vi "Dresden R2R Sputter 03.02.2018 IY24.vi"() -> ()   [LabVIEW 2009] (continued)
                                frame #0 {
                                n30316 = local write "SDC1 9"(TRUE ("SDC1 9")) -> ()
                                n30317 = Wait (ms)(milliseconds to wait=u32 1000) -> ()  [unwired: 1 out]
                                }
                                frame #1 {
                                }
                                }
                                }
                                }
                                }
                                }
                                }
                                frame #1 {
                                }
                                }
                                }
                                frame #11 {
                                n30318 = local read "Semi"() -> (w35192:bool)
                                n30319 = case shown="False" w35192 {
                                frame #0 {
                                n30320 = local write "Start_roll"(TRUE ("Start_roll")) -> ()
                                n30321 = Wait (ms)(milliseconds to wait=u32 300) -> ()  [unwired: 1 out]
                                }
                                frame #1 {
                                }
                                }
                                }
                                frame #12 {
                                n30322 = local read "Semi"() -> (w35195:bool)
                                n30323 = case shown="False" w35195 {
                                frame #0 {
                                n30324 = stacked-sequence {
                                frame #0 {
                                n30325 = local read "R Cmb Ch2 Step1 Coating Power Active"() -> (w35196:bool)
                                n30326 = case shown="True" w35196 {
                                frame #0 {
                                }
                                frame #1 {
                                n30327 = while {
                                stop <- w35198 stop-if-true
                                n30328 = local read "R Cmb Interval length"() -> (w35202:dbl)
                                n30329 = local read "Actual Length"() -> (w35201:dbl)
                                n30330 = Greater Or Equal?(x=w35201, y=w35202) -> (x >= y?=w35200:bool)
                                n30331 = local read "Semi"() -> (w35199:bool)
                                n30332 = Or(x=w35200, y=w35199) -> (x .or. y?=w35198:bool)
                                n30333 = Wait Until Next ms Multiple(millisecond multiple=u32 300) -> ()  [unwired: 1 out]
                                }
                                }
                                }
                                }
                                frame #1 {
                                n30334 = local read "R Cmb Ch2 Step2 Coating Power Active"() -> (w35203:bool)
                                n30335 = case shown="True" w35203 {
                                frame #0 {
                                }
                                frame #1 {
                                n30336 = stacked-sequence {
                                frame #0 {
                                n30337 = local read "Semi"() -> (w35204:bool)
                                n30338 = case shown="False" w35204 {
                                frame #0 {
                                n30339 = local read "R Cmb Ch3 Step2 Coating Power"() -> (w35206:dbl)
                                n30340 = Wait (ms)(milliseconds to wait=u32 200) -> ()  [unwired: 1 out]
                                n30341 = local write "Set DC Power       : 2"(w35206) -> ()
                                }
                                frame #1 {
                                }
                                }
                                }
                                frame #1 {
                                n30342 = local read "Semi"() -> (w35207:bool)
                                n30343 = case shown="False" w35207 {
                                frame #0 {
                                n30344 = local write "Dc_auto_set"(TRUE ("Dc_auto_set")) -> ()
                                }
                                frame #1 {
                                }
                                }
                                }
                                frame #2 {
                                n30345 = while {
                                stop <- w35213 stop-if-true
                                n30346 = local read "R Cmb Interval length"() -> (w35212:dbl)
                                n30347 = local read "Actual Length"() -> (w35216:dbl)
                                n30348 = Multiply(x=w35212, y=2.0) -> (x*y=w35210:dbl)
                                n30349 = Greater Or Equal?(x=w35216, y=w35210) -> (x >= y?=w35215:bool)
                                n30350 = local read "Semi"() -> (w35214:bool)
                                n30351 = Or(x=w35215, y=w35214) -> (x .or. y?=w35213:bool)
                                n30352 = Wait Until Next ms Multiple(millisecond multiple=u32 300) -> ()  [unwired: 1 out]
                                }
                                }
                                }
                                }
                                }
                                }
                                frame #2 {
                                n30353 = local read "R Cmb Ch2 Step3 Coating Power Active"() -> (w35217:bool)
                                n30354 = case shown="True" w35217 {
                                frame #0 {
                                }
                                frame #1 {
                                n30355 = stacked-sequence {
                                frame #0 {
                                n30356 = local read "Semi"() -> (w35218:bool)
                                n30357 = case shown="False" w35218 {
                                frame #0 {
                                n30358 = local read "R Cmb Ch3 Step3 Coating Power"() -> (w35220:dbl)
                                n30359 = Wait (ms)(milliseconds to wait=u32 200) -> ()  [unwired: 1 out]
                                n30360 = local write "Set DC Power       : 2"(w35220) -> ()
                                }
                                frame #1 {
                                }
                                }
                                }
                                frame #1 {
                                n30361 = local read "Semi"() -> (w35221:bool)
                                n30362 = case shown="False" w35221 {
                                frame #0 {
                                n30363 = local write "Dc_auto_set"(TRUE ("Dc_auto_set")) -> ()
                                }
                                frame #1 {
                                }
                                }
                                }
                                frame #2 {
                                n30364 = while {
                                stop <- w35227 stop-if-true
                                n30365 = local read "R Cmb Interval length"() -> (w35226:dbl)
                                n30366 = local read "Actual Length"() -> (w35230:dbl)
                                n30367 = Multiply(x=w35226, y=3.0) -> (x*y=w35224:dbl)
                                n30368 = Greater Or Equal?(x=w35230, y=w35224) -> (x >= y?=w35229:bool)
                                n30369 = local read "Semi"() -> (w35228:bool)
                                n30370 = Or(x=w35229, y=w35228) -> (x .or. y?=w35227:bool)
                                n30371 = Wait Until Next ms Multiple(millisecond multiple=u32 300) -> ()  [unwired: 1 out]
                                }
                                }
                                }
                                }
                                }
                                }
                                frame #3 {
                                n30372 = local read "R Cmb Ch2 Step4 Coating Power Active"() -> (w35231:bool)
                                n30373 = case shown="True" w35231 {
                                frame #0 {
                                }
                                frame #1 {
                                n30374 = stacked-sequence {
                                frame #0 {
                                n30375 = local read "Semi"() -> (w35232:bool)
                                n30376 = case shown="False" w35232 {
                                frame #0 {
                                n30377 = local read "R Cmb Ch3 Step4 Coating Power"() -> (w35234:dbl)
                                n30378 = Wait (ms)(milliseconds to wait=u32 200) -> ()  [unwired: 1 out]
                                n30379 = local write "Set DC Power       : 2"(w35234) -> ()
                                }
                                frame #1 {
                                }
                                }
                                }
                                frame #1 {
                                n30380 = local read "Semi"() -> (w35235:bool)
                                n30381 = case shown="False" w35235 {
                                frame #0 {
                                n30382 = local write "Dc_auto_set"(TRUE ("Dc_auto_set")) -> ()
                                }
                                frame #1 {
                                }
                                }
                                }
                                frame #2 {
                                n30383 = while {
                                stop <- w35241 stop-if-true
                                n30384 = local read "R Cmb Interval length"() -> (w35240:dbl)
                                n30385 = local read "Actual Length"() -> (w35244:dbl)
                                n30386 = Multiply(x=w35240, y=4.0) -> (x*y=w35238:dbl)
                                n30387 = Greater Or Equal?(x=w35244, y=w35238) -> (x >= y?=w35243:bool)
                                n30388 = local read "Semi"() -> (w35242:bool)
                                n30389 = Or(x=w35243, y=w35242) -> (x .or. y?=w35241:bool)
                                n30390 = Wait Until Next ms Multiple(millisecond multiple=u32 300) -> ()  [unwired: 1 out]
                                }
                                }
                                }
                                }
                                }
                                }
                                frame #4 {
                                n30391 = local read "R Cmb Ch2 Step5 Coating Power Active"() -> (w35245:bool)
                                n30392 = case shown="True" w35245 {
                                frame #0 {
                                }
                                frame #1 {
                                n30393 = stacked-sequence {
                                frame #0 {
                                n30394 = local read "Semi"() -> (w35246:bool)
                                n30395 = case shown="False" w35246 {
                                frame #0 {
                                n30396 = local read "R Cmb Ch3 Step5 Coating Power"() -> (w35248:dbl)
                                n30397 = Wait (ms)(milliseconds to wait=u32 200) -> ()  [unwired: 1 out]
                                n30398 = local write "Set DC Power       : 2"(w35248) -> ()
                                }
                                frame #1 {
                                }
                                }
                                }
                                frame #1 {
                                n30399 = local read "Semi"() -> (w35249:bool)
                                n30400 = case shown="False" w35249 {
                                frame #0 {
                                n30401 = local write "Dc_auto_set"(TRUE ("Dc_auto_set")) -> ()
                                }
                                frame #1 {
                                }
                                }
                                }
                                frame #2 {
                                n30402 = while {
                                stop <- w35255 stop-if-true
                                n30403 = local read "R Cmb Interval length"() -> (w35254:dbl)
                                n30404 = local read "Actual Length"() -> (w35258:dbl)
                                n30405 = Multiply(x=w35254, y=5.0) -> (x*y=w35252:dbl)
                                n30406 = Greater Or Equal?(x=w35258, y=w35252) -> (x >= y?=w35257:bool)
                                n30407 = local read "Semi"() -> (w35256:bool)
                                n30408 = Or(x=w35257, y=w35256) -> (x .or. y?=w35255:bool)
                                n30409 = Wait Until Next ms Multiple(millisecond multiple=u32 300) -> ()  [unwired: 1 out]
                                }
                                }
                                }
                                }
                                }
                                }
                                }
                                }
                                frame #1 {
                                }
                                }
                                }
                                frame #13 {
                                n30410 = local read "Semi"() -> (w35259:bool)
                                n30411 = case shown="False" w35259 {
                                frame #0 {
                                n30412 = local write "SDC1 13b"(TRUE ("SDC1 13b")) -> ()
                                n30413 = Wait (ms)(milliseconds to wait=u32 1000) -> ()  [unwired: 1 out]
                                }
                                frame #1 {
                                }
                                }
                                }
                                }
                                }
                                frame #14 {
                                # "CLOSE DC"
                                n30414 = local read "Semi"() -> (w35262:bool)
                                n30415 = case shown="False" w35262 {
                                frame #0 {
                                n30416 = stacked-sequence {
                                frame #0 {
                                n30417 = local read "Semi"() -> (w35263:bool)
                                n30418 = case shown="False" w35263 {
                                frame #0 {
                                n30419 = local write "Dc_auto_off"(TRUE ("Dc_auto_off")) -> ()
                                }
                                frame #1 {
                                }
                                }
                                }
                                frame #1 {
                                n30420 = local read "Semi"() -> (w35265:bool)
                                n30421 = case shown="False" w35265 {
                                frame #0 {
                                n30422 = Wait (ms)(milliseconds to wait=u32 1000) -> ()  [unwired: 1 out]
                                }
                                frame #1 {
                                }
                                }
                                }
                                frame #2 {
                                n30423 = local read "Semi"() -> (w35267:bool)
                                n30424 = case shown="False" w35267 {
                                frame #0 {
                                n30425 = local write "Dc_auto_set_zero"(TRUE ("Dc_auto_set")) -> ()
                                }
                                frame #1 {
                                }
                                }
                                }
                                frame #3 {
                                n30426 = local read "Semi"() -> (w35269:bool)
                                n30427 = case shown="False" w35269 {
                                frame #0 {
                                n30428 = Wait (ms)(milliseconds to wait=u32 1000) -> ()  [unwired: 1 out]
                                }
                                frame #1 {
                                }
                                }
                                }
                                frame #4 {
                                n30429 = local read "Semi"() -> (w35271:bool)
                                n30430 = case shown="False" w35271 {
                                frame #0 {
                                n30431 = while {
                                i -> [w35283]
                                stop <- w35272 stop-if-true
                                n30432 = Greater?(x=w35283, y=600) -> (0:w35282:bool)
                                n30433 = case shown="True" w35282 {
                                frame #0 {
                                }
                                frame #1 {
                                n30434 = local write "Semi"(TRUE ("Semi")) -> ()
                                n30435 = local write "Error Message"("Sputter Process cancelled.\nPlease Check DC connections." ("Error Message")) -> ()
                                }
                                }
                                n30436 = local read "Actual DC Power : 2"() -> (w35277:dbl)
                                n30437 = local read "Actual DC Volt2"() -> (w35276:dbl)
                                n30438 = Less?(x=w35277, y=10.0) -> (x < y?=w35280:bool)
                                n30439 = Less?(x=w35276, y=20.0) -> (x < y?=w35281:bool)
                                n30440 = And(x=w35280, y=w35281) -> (x .and. y?=w35274:bool)
                                n30441 = local read "Semi"() -> (w35273:bool)
                                n30442 = Wait Until Next ms Multiple(millisecond multiple=u32 500) -> ()  [unwired: 1 out]
                                n30443 = Compound Arithmetic op=OR(w35274, w35273) -> (w35272:bool)
                                }
                                }
                                frame #1 {
                                }
                                }
                                }
                                frame #5 {
                                n30444 = local read "Semi"() -> (w35287:bool)
                                n30445 = case shown="False" w35287 {
                                frame #0 {
                                n30446 = while {
                                i -> [w35293]
                                stop <- w35288 stop-if-true
                                n30447 = Greater?(x=w35293, y=50) -> (0:w35292:bool)
                                n30448 = case shown="True" w35292 {
                                frame #0 {
                                }
                                frame #1 {
                                n30449 = local write "Semi"(TRUE ("Semi")) -> ()
                                n30450 = local write "Error Message"("Sputter Process cancelled.\nPlease Check DCPS-SW2." ("Error Message")) -> ()
                                }
                                }
                                n30451 = local read "Cnt_Dcps_sw2_di"() -> (w35291:bool)
                                n30452 = case shown="True" w35291 {
                                tunnel: [TRUE ("Cnt_Dcps_sw1_do") FALSE ("Cnt_Dcps_sw1_do")] -> w35290
                                frame #0 {
                                }
                                frame #1 {
                                n30453 = local write "Cnt_Dcps_sw2_do"(FALSE ("Cnt_Dcps_sw1_do")) -> ()
                                n30454 = Wait Until Next ms Multiple(millisecond multiple=u32 500) -> ()  [unwired: 1 out]
                                }
                                }
                                n30455 = local read "Semi"() -> (w35289:bool)
                                n30456 = Or(x=w35290, y=w35289) -> (x .or. y?=w35288:bool)
                                }
                                }
                                frame #1 {
                                }
                                }
                                }
                                frame #6 {
                                n30457 = local read "Semi"() -> (w35301:bool)
                                n30458 = case shown="False" w35301 {
                                frame #0 {
                                n30459 = Wait (ms)(milliseconds to wait=u32 1000) -> ()  [unwired: 1 out]
                                n30460 = local write "SDC1 25"(TRUE ("SDC1 25")) -> ()
                                }
                                frame #1 {
                                }
                                }
                                }
                                }
                                }
                                frame #1 {
                                }
                                }
                                }
                                frame #15 {
                                # "PC-BV OPEN"
                                n30461 = stacked-sequence {
                                frame #0 {
                                n30462 = local read "Semi"() -> (w35304:bool)
                                n30463 = case shown="False" w35304 {
                                frame #0 {
                                n30464 = stacked-sequence {
                                frame #0 {
                                n30465 = local read "Semi"() -> (w35305:bool)
                                n30466 = case shown="False" w35305 {
                                frame #0 {
                                n30467 = local write "Pc_bv3_auto_open"(TRUE ("Tp1_auto_start")) -> ()
                                }
                                frame #1 {
                                }
                                }
                                }
                                frame #1 {
                                n30468 = local read "Semi"() -> (w35307:bool)
                                n30469 = case shown="False" w35307 {
                                frame #0 {
                                n30470 = Wait (ms)(milliseconds to wait=u32 1000) -> ()  [unwired: 1 out]
                                }
                                frame #1 {
                                }
                                }
                                }
                                frame #2 {
                                n30471 = local read "Semi"() -> (w35309:bool)
                                n30472 = case shown="False" w35309 {
                                frame #0 {
                                n30473 = while {
                                i -> [w35315]
                                stop <- w35311 stop-if-true
                                n30474 = local read "Pc_bv_opened_ch3"() -> (w35313:bool)
                                n30475 = Greater?(x=w35315, y=120) -> (0:w35314:bool)
                                n30476 = local read "Semi"() -> (w35312:bool)
                                n30477 = Compound Arithmetic op=OR(w35312, w35313, w35314) -> (w35311:bool)
                                n30478 = Wait (ms)(milliseconds to wait=u32 500) -> ()  [unwired: 1 out]
                                }
                                }
                                frame #1 {
                                }
                                }
                                }
                                frame #3 {
                                n30479 = local read "Semi"() -> (w35317:bool)
                                n30480 = case shown="False" w35317 {
                                frame #0 {
                                n30481 = local read "Pc_bv_opened_ch3"() -> (w35318:bool)
                                n30482 = case shown="False" w35318 {
                                frame #0 {
                                n30483 = local write "Pc_bv3_auto_open"(TRUE ("Pc_bv1_auto_open")) -> ()
                                }
                                frame #1 {
                                }
                                }
                                }
                                frame #1 {
                                }
                                }
                                }
                                frame #4 {
                                n30484 = local read "Semi"() -> (w35320:bool)
                                n30485 = case shown="False" w35320 {
                                frame #0 {
                                n30486 = local read "Pc_bv_opened_ch3"() -> (w35321:bool)
                                n30487 = case shown="False" w35321 {
                                frame #0 {
                                n30488 = Wait (ms)(milliseconds to wait=u32 1000) -> ()  [unwired: 1 out]
                                }
                                frame #1 {
                                }
                                }
                                }
                                frame #1 {
                                }
                                }
                                }
                                frame #5 {
                                n30489 = local read "Semi"() -> (w35323:bool)
                                n30490 = case shown="False" w35323 {
                                frame #0 {
                                n30491 = while {
                                i -> [w35329]
                                stop <- w35325 stop-if-true
                                n30492 = local read "Pc_bv_opened_ch3"() -> (w35327:bool)
                                n30493 = Greater?(x=w35329, y=120) -> (0:w35328:bool)
                                n30494 = local read "Semi"() -> (w35326:bool)
                                n30495 = Compound Arithmetic op=OR(w35326, w35327, w35328) -> (w35325:bool)
                                n30496 = Wait (ms)(milliseconds to wait=u32 500) -> ()  [unwired: 1 out]
                                }
                                }
                                frame #1 {
                                }
                                }
                                }
                                frame #6 {
                                n30497 = local read "Semi"() -> (w35331:bool)
                                n30498 = case shown="False" w35331 {
                                frame #0 {
                                n30499 = local read "Pc_bv_opened_ch3"() -> (w35332:bool)
                                n30500 = case shown="False" w35332 {
                                frame #0 {
                                n30501 = local write "Error Message"("Start up process  cancelled\nbecause  PC-BV not opened.\nPlease check PC-BV1 connections." ("Error Message")) -> ()
                                n30502 = Wait (ms)(milliseconds to wait=u32 1000) -> ()  [unwired: 1 out]
                                }
                                frame #1 {
                                }
                                }
                                }
                                frame #1 {
                                }
                                }
                                }
                                }
                                }
                                frame #1 {
                                }
                                }
                                }
                                frame #1 {
                                n30503 = local read "Semi"() -> (w35335:bool)
                                n30504 = case shown="False" w35335 {
                                frame #0 {
                                n30505 = Wait (ms)(milliseconds to wait=u32 1000) -> ()  [unwired: 1 out]
                                n30506 = local write "SDC1 28"(TRUE ("SDC1 28")) -> ()
                                }
                                frame #1 {
                                }
                                }
                                }
                                }
                                }
                                frame #16 {
                                # "set ar zero"
                                n30507 = stacked-sequence {
                                frame #0 {
                                n30508 = local read "Semi"() -> (w35338:bool)
                                n30509 = case shown="False" w35338 {
                                frame #0 {
                                n30510 = stacked-sequence {
                                frame #0 {
                                n30511 = local read "Semi"() -> (w35339:bool)
                                n30512 = case shown="False" w35339 {
                                frame #0 {
                                n30513 = local write "Ar_auto_set_zero_ch3"(TRUE ("Ar_auto_set_zero_ch1")) -> ()
                                }
                                frame #1 {
                                }
                                }
                                }
                                frame #1 {
                                n30514 = local read "Semi"() -> (w35341:bool)
                                n30515 = case shown="False" w35341 {
                                frame #0 {
                                n30516 = while {
                                i -> [w35344]
                                stop <- w35343 stop-if-true
                                n30517 = Greater?(x=w35344, y=150) -> (0:w35343:bool)
                                n30518 = local read "Semi"() -> (w35342:bool)
                                n30519 = case shown="False" w35342 {
                                tunnel: [FALSE TRUE] -> _
                                frame #0 {
                                n30520 = Wait Until Next ms Multiple(millisecond multiple=u32 200) -> ()  [unwired: 1 out]
                                }
                                frame #1 {
                                }
                                }
                                }
                                }
                                frame #1 {
                                }
                                }
                                }
                                frame #2 {
                                n30521 = local read "Semi"() -> (w35349:bool)
                                n30522 = case shown="False" w35349 {
                                frame #0 {
                                n30523 = local read "Ar_sccm_act 2"() -> (w35350:dbl)
                                n30524 = Less?(x=w35350, y=1) -> (x < y?=w35351:bool)
                                n30525 = case shown="False" w35351 {
                                frame #0 {
                                n30526 = local write "Ar_auto_set_zero_ch3"(TRUE ("Ar_auto_set_zero_ch1")) -> ()
                                }
                                frame #1 {
                                }
                                }
                                }
                                frame #1 {
                                }
                                }
                                }
                                frame #3 {
                                n30527 = local read "Semi"() -> (w35354:bool)
                                n30528 = case shown="False" w35354 {
                                frame #0 {
                                n30529 = local read "Ar_sccm_act 2"() -> (w35355:dbl)
                                n30530 = Less?(x=w35355, y=1) -> (x < y?=w35356:bool)
                                n30531 = case shown="False" w35356 {
                                frame #0 {
                                n30532 = while {
                                i -> [w35362]
                                stop <- w35359 stop-if-true
                                n30533 = Greater?(x=w35362, y=150) -> (0:w35360:bool)
                                n30534 = local read "Semi"() -> (w35358:bool)
                                n30535 = case shown="True" w35358 {
                                tunnel: [FALSE FALSE] -> w35361
                                frame #0 {
                                }
                                frame #1 {
                                n30536 = Wait Until Next ms Multiple(millisecond multiple=u32 200) -> ()  [unwired: 1 out]
                                }
                                }
                                n30537 = Or(x=w35361, y=w35360) -> (x .or. y?=w35359:bool)
                                }
                                }
                                frame #1 {
                                }
                                }
                                }
                                frame #1 {
                                }
                                }
                                }
                                frame #4 {
                                n30538 = local read "Semi"() -> (w35367:bool)
                                n30539 = case shown="False" w35367 {
                                frame #0 {
                                n30540 = Wait (ms)(milliseconds to wait=u32 1000) -> ()  [unwired: 1 out]
                                }
                                frame #1 {
                                }
                                }
                                }
                                }
                                }
                                frame #1 {
                                }
                                }
                                }
                                frame #1 {
                                n30541 = local read "Semi"() -> (w35369:bool)
                                n30542 = case shown="False" w35369 {
                                frame #0 {
                                n30543 = local write "SDC1 26"(TRUE ("SDC1 26")) -> ()
                                n30544 = Wait (ms)(milliseconds to wait=u32 1000) -> ()  [unwired: 1 out]
                                }
                                frame #1 {
                                }
                                }
                                }
                                }
                                }
                                frame #17 {
                                # "sov-ar close"
                                n30545 = stacked-sequence {
                                frame #0 {
                                n30546 = local read "Semi"() -> (w35372:bool)
                                n30547 = case shown="False" w35372 {
                                frame #0 {
                                n30548 = while {
                                i -> [w35378]
                                stop <- w35373 stop-if-true
                                n30549 = Greater?(x=w35378, y=50) -> (0:w35377:bool)
                                n30550 = case shown="True" w35377 {
                                frame #0 {
                                }
                                frame #1 {
                                n30551 = local write "Semi"(TRUE ("Semi")) -> ()
                                n30552 = local write "Error Message"("Coating Process  \nwas cancelled.\nPlease check \nSOV-Ar connection." ("Error Message")) -> ()
                                }
                                }
                                n30553 = local read "Ch3_Sov_Ar_di"() -> (w35376:bool)
                                n30554 = case shown="True" w35376 {
                                tunnel: [TRUE FALSE] -> w35375
                                frame #0 {
                                }
                                frame #1 {
                                n30555 = local write "Ch3_Sov_Ar_do"(FALSE ("Ch1_WFC_do")) -> ()
                                n30556 = Wait Until Next ms Multiple(millisecond multiple=u32 200) -> ()  [unwired: 1 out]
                                }
                                }
                                n30557 = local read "Semi"() -> (w35374:bool)
                                n30558 = Or(x=w35375, y=w35374) -> (x .or. y?=w35373:bool)
                                }
                                }
                                frame #1 {
                                }
                                }
                                }
                                frame #1 {
                                n30559 = local read "Semi"() -> (w35386:bool)
                                n30560 = case shown="False" w35386 {
                                frame #0 {
                                n30561 = local write "SDC1 27"(TRUE ("SDC1 27")) -> ()
                                n30562 = Wait (ms)(milliseconds to wait=u32 1000) -> ()  [unwired: 1 out]
                                }
                                frame #1 {
                                }
                                }
                                }
                                }
                                }
                                frame #18 {
                                # "CC OPEN"
                                n30563 = stacked-sequence {
                                frame #0 {
                                n30564 = local read "Semi"() -> (w35389:bool)
                                n30565 = case shown="False" w35389 {
                                frame #0 {
                                n30566 = while {
                                i -> [w35395]
                                stop <- w35390 stop-if-true
                                n30567 = Greater?(x=w35395, y=50) -> (0:w35394:bool)
                                n30568 = case shown="True" w35394 {
                                frame #0 {
                                }
                                frame #1 {
                                n30569 = local write "Semi"(TRUE ("Semi")) -> ()
                                n30570 = local write "Error Message"("Coating Process  \nwas cancelled.\nPlease check \nBG-BV connection." ("Error Message")) -> ()
                                }
                                }
                                n30571 = local read "Ch3_Cc_on_off_di"() -> (w35393:bool)
                                n30572 = case shown="False" w35393 {
                                tunnel: [FALSE TRUE] -> w35392
                                frame #0 {
                                n30573 = local write "Ch3_Cc_on_off_do"(TRUE ("Ch1_WFC_do")) -> ()
                                n30574 = Wait Until Next ms Multiple(millisecond multiple=u32 200) -> ()  [unwired: 1 out]
                                }
                                frame #1 {
                                }
                                }
                                n30575 = local read "Semi"() -> (w35391:bool)
                                n30576 = Or(x=w35392, y=w35391) -> (x .or. y?=w35390:bool)
                                }
                                }
                                frame #1 {
                                }
                                }
                                }
                                frame #1 {
                                n30577 = local read "Semi"() -> (w35403:bool)
                                n30578 = case shown="False" w35403 {
                                frame #0 {
                                n30579 = while {
                                i -> [w35408]
                                stop <- w35406 stop-if-true
                                n30580 = Greater?(x=w35408, y=30) -> (0:w35404:bool)
                                n30581 = Wait Until Next ms Multiple(millisecond multiple=u32 1000) -> ()  [unwired: 1 out]
                                n30582 = local read "Semi"() -> (w35407:bool)
                                n30583 = Or(x=w35404, y=w35407) -> (x .or. y?=w35406:bool)
                                }
                                }
                                frame #1 {
                                }
                                }
                                }
                                frame #2 {
                                n30584 = local read "Semi"() -> (w35410:bool)
                                n30585 = case shown="False" w35410 {
                                frame #0 {
                                n30586 = local write "SDC1 27b"(TRUE ("SDC1 3")) -> ()
                                n30587 = Wait (ms)(milliseconds to wait=u32 1000) -> ()  [unwired: 1 out]
                                }
                                frame #1 {
                                }
                                }
                                }
                                }
                                }
                                frame #19 {
                                # "CHECK CHAMBER PRESSURE"
                                n30588 = stacked-sequence {
                                frame #0 {
                                n30589 = local read "Semi"() -> (w35413:bool)
                                n30590 = case shown="False" w35413 {
                                frame #0 {
                                n30591 = while {
                                i -> [w35421]
                                stop <- w35415 stop-if-true
                                n30592 = Greater?(x=w35421, y=300) -> (0:w35420:bool)
                                n30593 = case shown="True" w35420 {
                                frame #0 {
                                }
                                frame #1 {
                                n30594 = local write "Semi"(TRUE ("Semi")) -> ()
                                n30595 = local write "Error Message"("Coating Process cancelled.\nPlease check chamber \nconnections." ("Error Message")) -> ()
                                }
                                }
                                n30596 = local read "Ch_CC_press_ch3 2"() -> (w35414:dbl)
                                n30597 = Greater Or Equal?(x=w35414, y=5e-05 ("CHAMBER PRESSURE 6")) -> (x >= y?=w35418:bool)
                                n30598 = case shown="True" w35418 {
                                tunnel: [TRUE FALSE] -> w35417
                                frame #0 {
                                }
                                frame #1 {
                                n30599 = Wait Until Next ms Multiple(millisecond multiple=u32 200) -> ()  [unwired: 1 out]
                                }
                                }
                                n30600 = local read "Semi"() -> (w35416:bool)
                                n30601 = Or(x=w35417, y=w35416) -> (x .or. y?=w35415:bool)
                                }
                                }
                                frame #1 {
                                }
                                }
                                }
                                frame #1 {
                                n30602 = local read "Semi"() -> (w35428:bool)
                                n30603 = case shown="False" w35428 {
                                frame #0 {
                                n30604 = Wait (ms)(milliseconds to wait=u32 1000) -> ()  [unwired: 1 out]
                                n30605 = local write "SDC1 27c"(TRUE ("SDC1 10")) -> ()
                                }
                                frame #1 {
                                }
                                }
                                }
                                }
                                }
                                frame #20 {
                                n30606 = local read "Semi"() -> (w35431:bool)
                                n30607 = case shown="False" w35431 {
                                frame #0 {
                                n30608 = Wait (ms)(milliseconds to wait=u32 1000) -> ()  [unwired: 1 out]
                                n30609 = local write "SDC1 30"(TRUE ("SDC1 30")) -> ()
                                }
                                frame #1 {
                                }
                                }
                                }
                                }
                                }